vi "ScanDelay_FTIR_BBnorm_Aligning.vi"() -> ()   [LabVIEW 2021]
uses:
  Control_scanDelayWorkflow.ctl
  Control_GetSpectrum_BBnorm.ctl
  C:/Users/mnopl/Desktop/Software/mnOPSuite/PRISM/Thorlabs.MotionControl.FilterFlipperCLI.dll
  Thorlabs.MotionControl.FilterFlipperCLI.dll
  C:/Users/mnopl/Desktop/Software/mnOPSuite/PRISM/Thorlabs.MotionControl.Controls.dll
  Thorlabs.MotionControl.Controls.dll
panel:
  in  "Realign phase":bool
  in  "Recalibrate BB\nfrequency":bool
  in  "Pause\nacquisition":bool
  in  "Replicate\nfrom #":i8=2 min=0
  in  "Envelope width":dbl(slide)=1.0454545454545454 scale=0.25..4.0
  out "Accumulated sample BB spectrum":dbl[][](array[numeric])
  out "Accumulated sample spectrum":dbl[][](array[numeric])
  in  "BB-reference spectrum":bool
  in  "Acquire only\nBB 100% curve with spoofed flip":bool
  in  "Acquire only\nBB 100% curve":bool
  in  "Toggle pause (ms)":dbl=500.0
  out "BB-referenced spectrum (phase)":T1(graph)
  out "BB-referenced spectrum (amplitude)":T2(graph)
  out "Reference BB spectra":dbl[][](array[numeric])
  out "Reference spectra":dbl[][](array[numeric])
  out "Latest replication cmd":string="@rep load 2"
  in  "Replicate\nalpha on\naccumulation":bool=TRUE
  out "# Accumulated":i32
  in  "Accumulate to #":i32=10
  in  "Cancel\nacquisition":bool
  out "Toggle position":i32=1
  in  "BB flipper serial #":string="37005305"
  in  "FilterFlipperControl":refnum<k24>(container)
  out "Spectrum stored":bool
  out "Reference stored":bool=TRUE
  out "Normalized spectrum (phase)":T1(graph)
  out "Normalized spectrum (amplitude)":T1(graph)
  in  "Store as reference":bool
  out "Python alpha rep path":path=path "C:/Users/mnopl/Desktop/Software/python/alpha/rep.py"
  out "Activity status":string="Awaiting command"
  out "Acquisition status":string="Ready to acquire spectrum"
  in  "Path to save spectrum":path=path "C:/Users/mnopl/Desktop/Software/LabVIEW/ScanDelay/Test Data/Ref spectra - silicon 1.txt"
  in  "Load reference":bool
  in  "Path to load reference":path=path "C:/Users/mnopl/Desktop/Software/LabVIEW/ScanDelay/Test Data/Ref spectra - silicon 1.txt"
  in  "Path to load spectrum":path=path "C:/Users/mnopl/Desktop/Software/LabVIEW/ScanDelay/Test Data/Sample spectra - sio2 100 nm.txt"
  in  "Apply spectral\nenvelope":bool=TRUE
  out "Binned interferogram":cluster{"X":dbl, "Y":dbl}[](graph)
  out "Sample BB Spectra":dbl[][](array[numeric])
  out "Sample Spectra":dbl[][](array[numeric])
  out "Python error: spectrum acquisition":errorcluster
  out "Python scandelay path":path=path "C:/Users/mnopl/Desktop/Software/LabVIEW/ScanDelay/scandelay.py"
  in  "Time per\nacquisition (s)":dbl=0.235
  in  "Sampling rate":dbl=250000.0
  in  "Delay calibratior\nfactor (ps/V)":dbl=2.403 format="%_6g"
  in  "Cycles per\ninterferogram":i32=80
  out "Python error: DAQ acquisition":errorcluster
  out "Accumulated spectrum (amplitude)":T3(graph)
  out "Acquisition cycle":dbl[][](graph)
  out "% averaged":dbl=100.0
  in  "Halt program":bool=TRUE
  out "Python error: activity loop":errorcluster
  in  "Load spectrum":bool
  in  "Save spectrum":bool
  in  "Normalize spectrum":bool
  in  "Acquire spectrum":bool
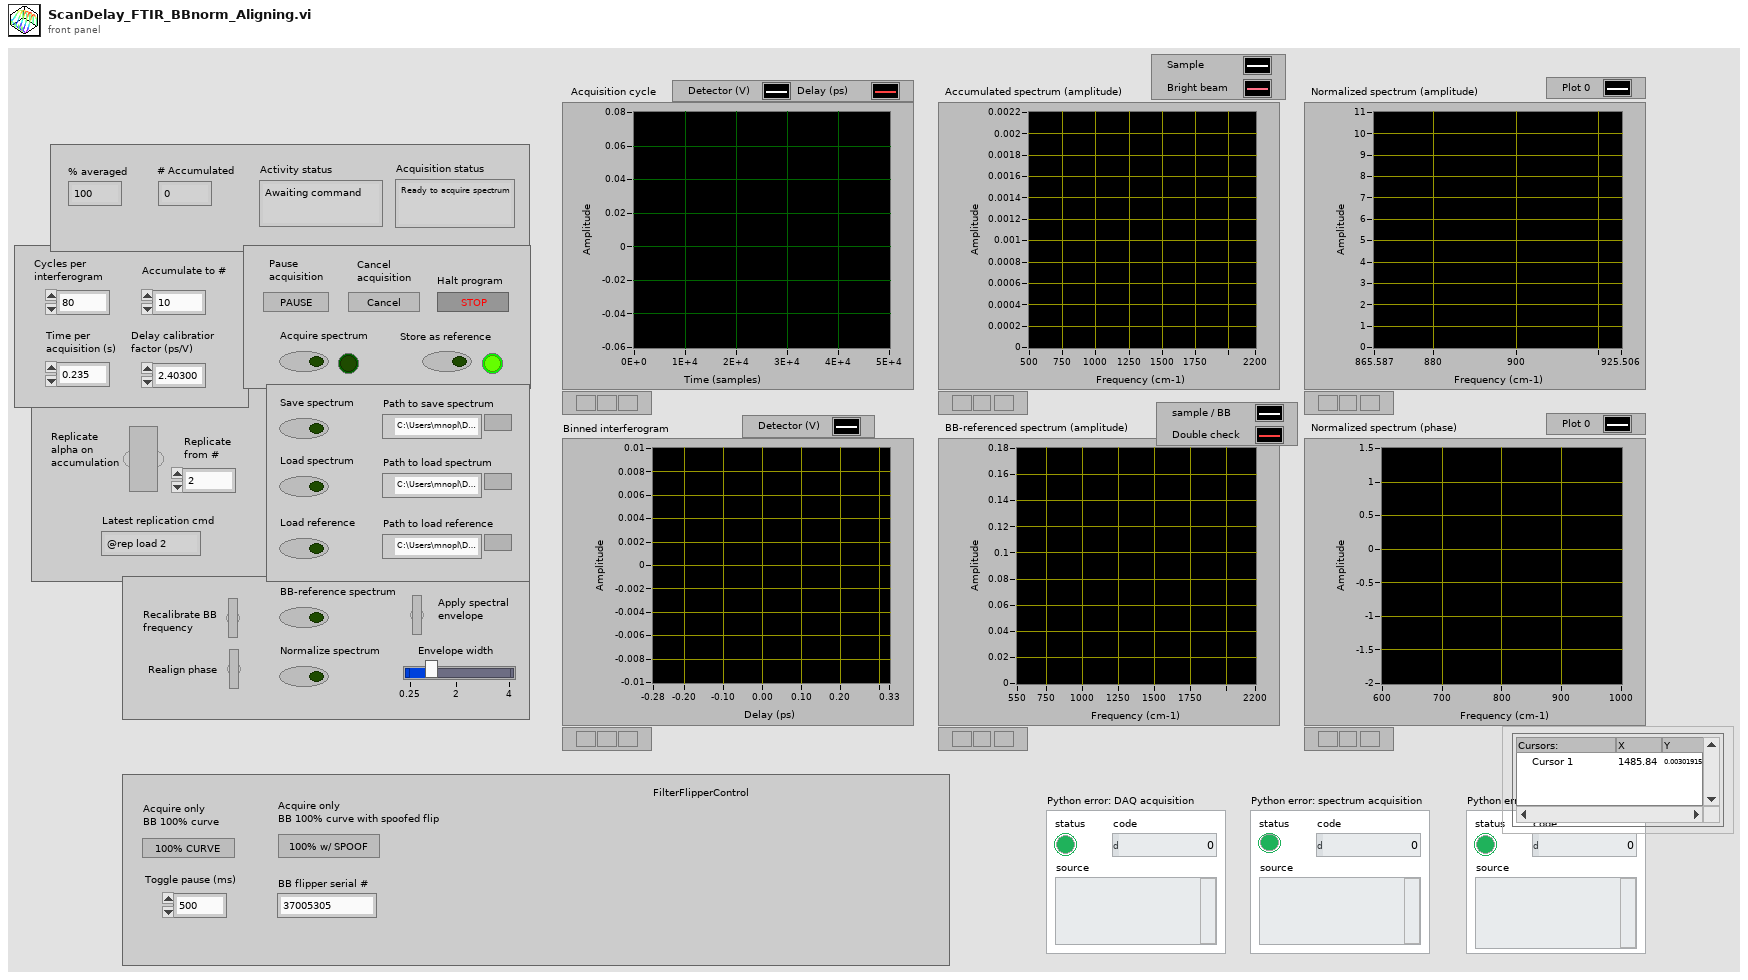
[diagram p1: front panel]
types:
  T1 = cluster{"Output spectrum":dbl[], "Output spectrum":dbl[]}
  T2 = cluster{"Sample Spectra":dbl[], "Sample Spectra":dbl[]}
  T3 = cluster{"Output spectrum":dbl[], "Output spectrum":dbl[]}[]
  T4 = typedef "Control_scanDelayWorkflow.ctl" = enum16{"Initialize", "Sit Idle", "Load Spectrum", "Store reference", "Save Spectrum", "Load reference", "Check Reference", "Check Spectrum", "BB reference spectrum", "Normalize Spectrum", "Done"}
  T5 = typedef "Control_GetSpectrum_BBnorm.ctl" = enum16{"Initialize", "Replicate alpha", "Flip in BB", "Get Spectrum", "Accumulate BB spectrum", "Flip out BB", "Accumulate sample spectrum", "Assess accumulation", "Finalize", "Done"}
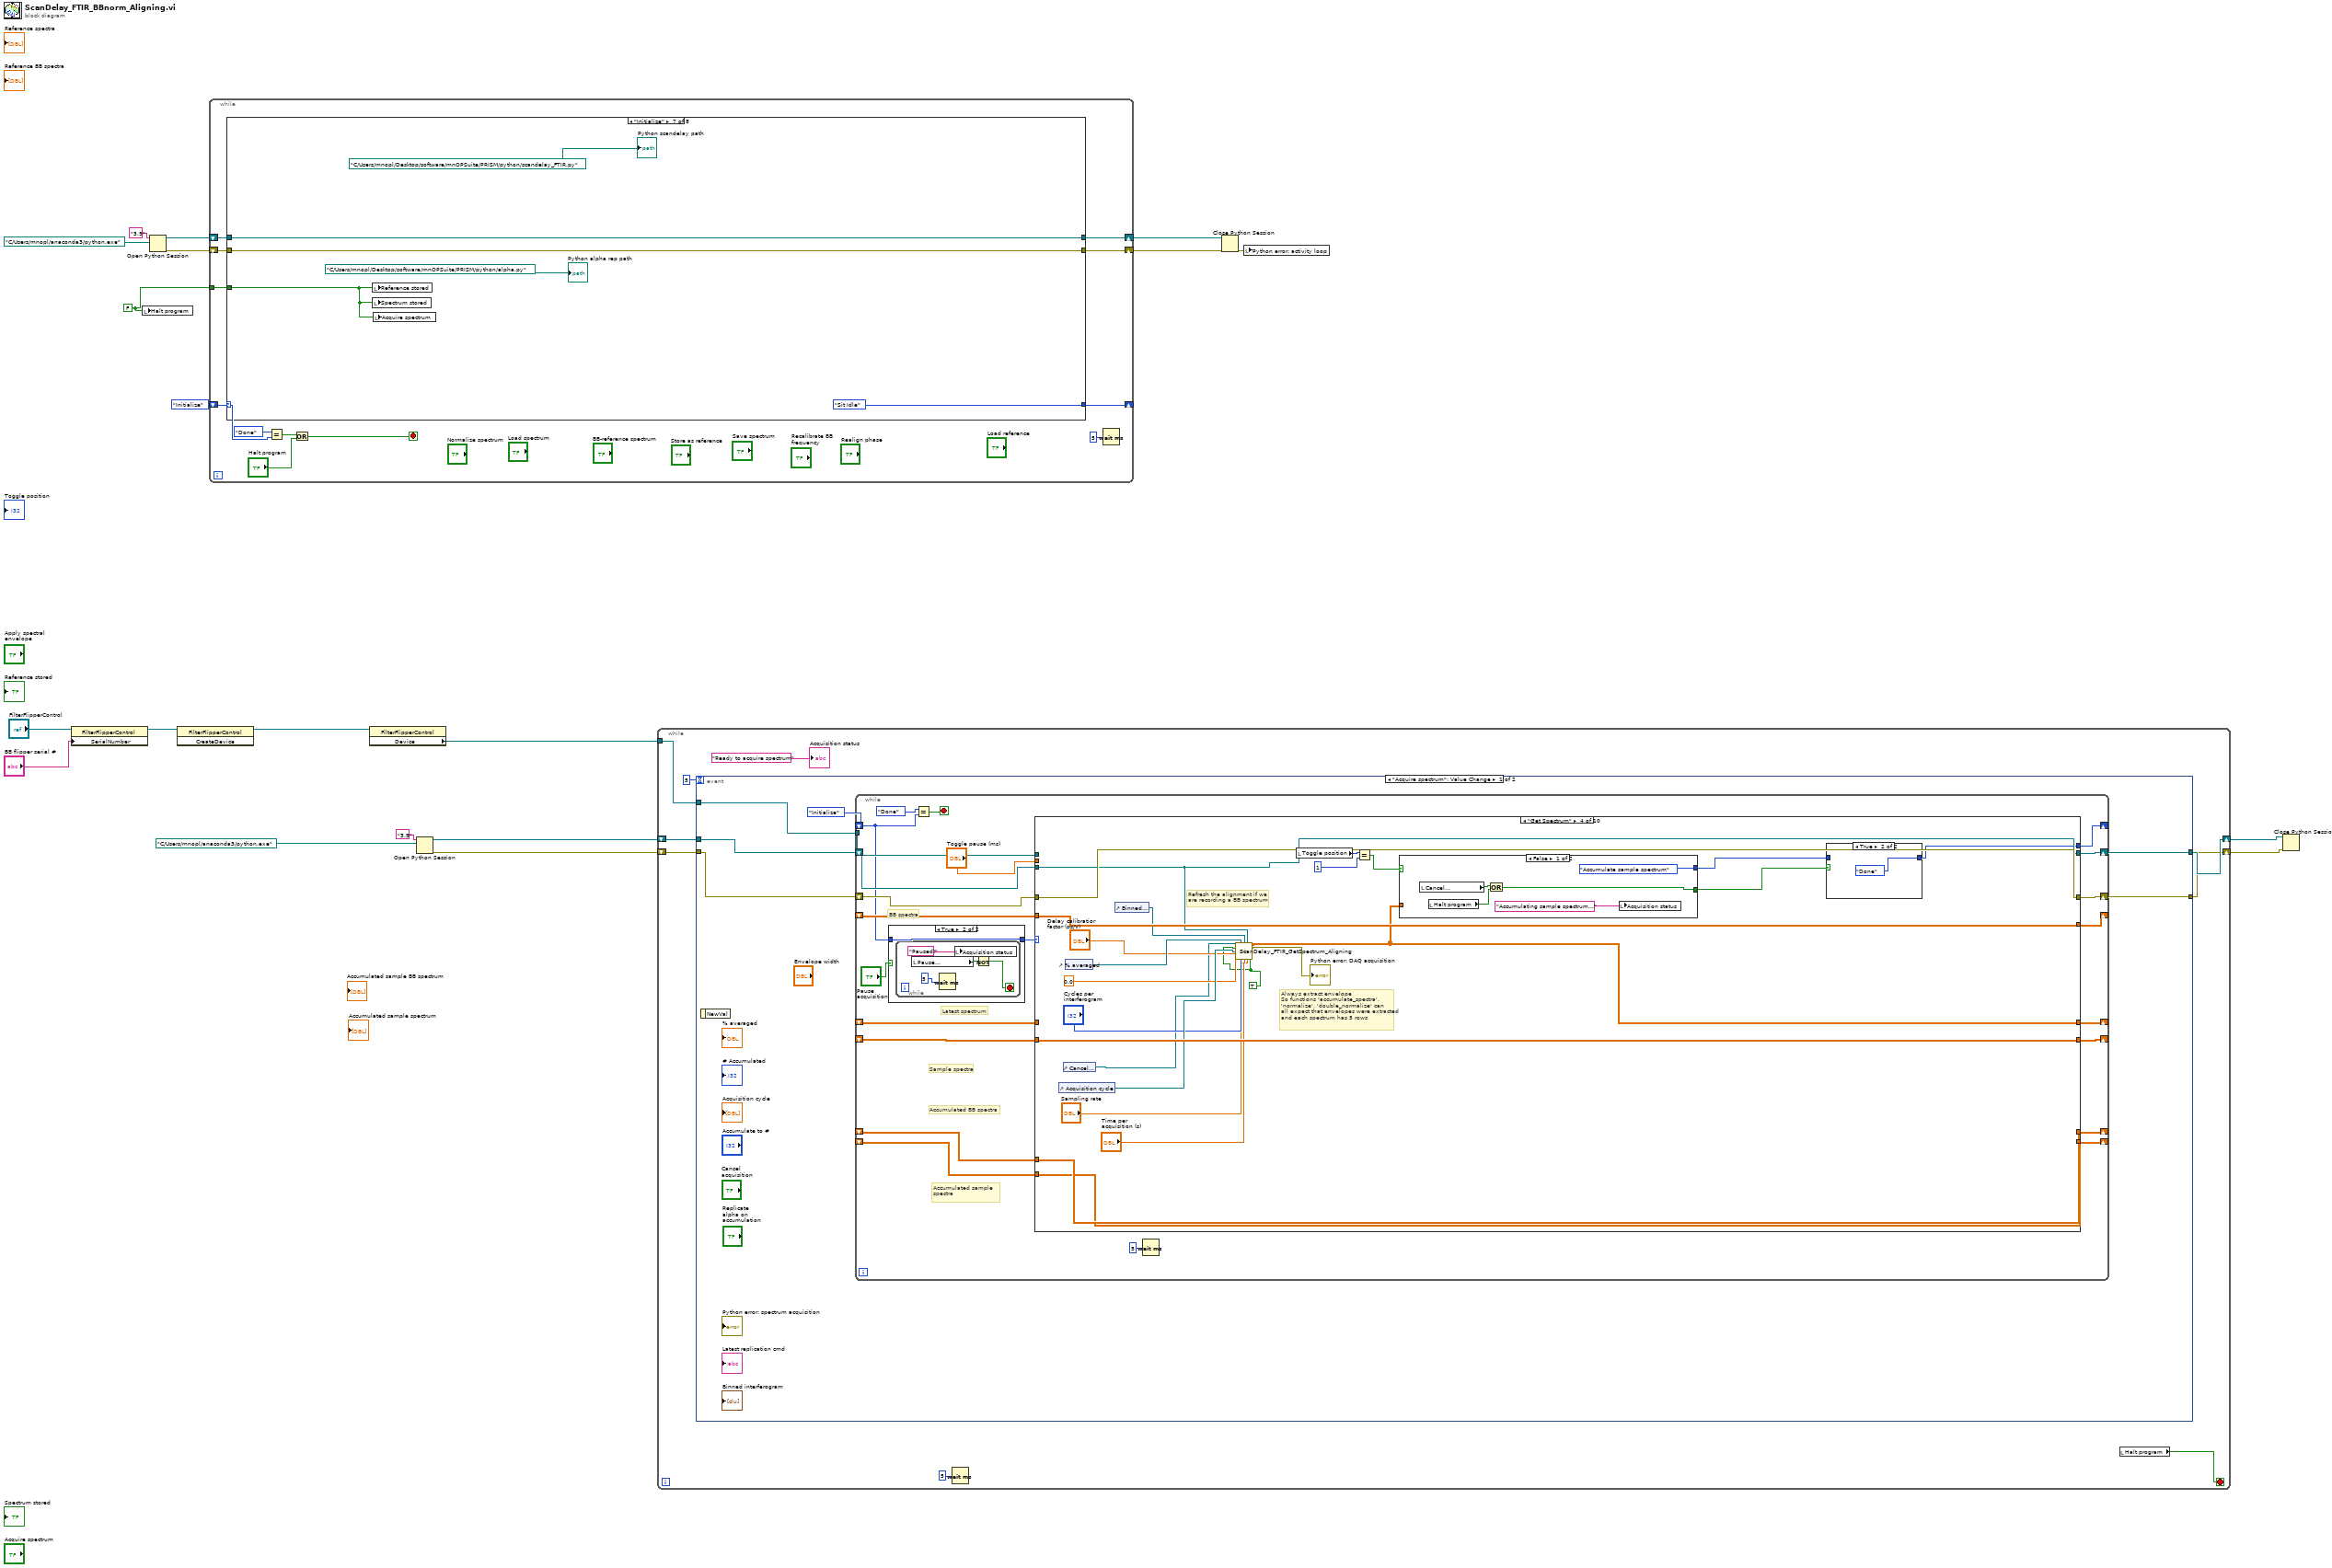
[diagram p0: block diagram]
diagram:
  w1 = FALSE
  n1 = property class="FilterFlipperControl"(reference="FilterFlipperControl", "SerialNumber"="BB flipper serial #") -> (reference out=w11:refnum<k24>)  [unwired: 1 in, 1 out]
  n2 = local write "Halt program"(w1) -> ()
  n3 = Open Python Session(python version="3.9", python path=path "C:/Users/mnopl/anaconda3/python.exe") -> (session out=w16:refnum<k35>, error out=w15:errorcluster)  [unwired: 1 in]
  n4 = invoke class="FilterFlipperControl" method="CreateDevice"(reference=w11) -> (reference out=w10:refnum<k24>)  [unwired: 2 in, 2 out]
  n5 = while {
    shift-right: [w25] -> _
    shift-left: Control_scanDelayWorkflow."Initialize" -> [w22]
    shift-right: [w31] -> w17
    shift-left: w15 -> [w23]
    shift-right: [w26] -> w18
    shift-left: w16 -> [w24]
    tunnel: w1 -> [w21]
    stop <- w29 stop-if-true
    n6 = case shown="\"Initialize\"" w22 {
      tunnel: [w36 w70 w80 w99 w120 w165 w184 w196] -> w31
      tunnel: w24 -> [w37 w69 w79 w100 w123 w166 w185 w194]
      tunnel: w23 -> [w36 w70 w80 w99 w122 w165 w184 w193]
      tunnel: [w37 w69 w79 w100 w121 w166 w185 w195] -> w26
      tunnel: [w35 Control_scanDelayWorkflow."Sit Idle" Control_scanDelayWorkflow."Sit Idle" Control_scanDelayWorkflow."Sit Idle" Control_scanDelayWorkflow."Sit Idle" Control_scanDelayWorkflow."Sit Idle" Control_scanDelayWorkflow."Sit Idle" Control_scanDelayWorkflow."Sit Idle"] -> w25
      tunnel: w21 -> [_ _ _ _ _ _ w181 _]
      frame "Sit Idle", Default {
        n7 = event shown="[2] \"BB-reference spectrum\": Value Change" {
          selector: _ -> [_ _ _ _ _ _ _]
          dyn-events: _ -> [_ _ _ _ _ _ _]
          timeout: 5 -> [_ _ _ _ _ _ w62]
          tunnel: [w38 w42 w49 w50 w54 w58 Control_scanDelayWorkflow."Sit Idle"] -> w35
          event "Normalize spectrum": Value Change {
            n8 = event-data() -> ("NewVal"=w39:bool)  [unwired: 1 in]
            n9 = Select(t=Control_scanDelayWorkflow."Normalize Spectrum", s=w39, f=Control_scanDelayWorkflow."Sit Idle") -> (s? t:f=w38:T4)
          }
          event "Store as reference": Value Change {
            n10 = event-data() -> ("NewVal"=w45:bool)  [unwired: 1 in]
            n11 = Select(t=Control_scanDelayWorkflow."Store reference", s=w45, f=Control_scanDelayWorkflow."Sit Idle") -> (s? t:f=w42:T4)
          }
          event "BB-reference spectrum": Value Change {
            n12 = event-data() -> ("NewVal"=w47:bool)  [unwired: 1 in]
            n13 = Select(t=Control_scanDelayWorkflow."BB reference spectrum", s=w47, f=Control_scanDelayWorkflow."Sit Idle") -> (s? t:f=w49:T4)
          }
          event "Save spectrum": Value Change {
            n14 = event-data() -> ("NewVal"=w51:bool)  [unwired: 1 in]
            n15 = Select(t=Control_scanDelayWorkflow."Save Spectrum", s=w51, f=Control_scanDelayWorkflow."Sit Idle") -> (s? t:f=w50:T4)
          }
          event "Load reference": Value Change {
            n16 = event-data() -> ("NewVal"=w57:bool)  [unwired: 1 in]
            n17 = Select(t=Control_scanDelayWorkflow."Load reference", s=w57, f=Control_scanDelayWorkflow."Sit Idle") -> (s? t:f=w54:T4)
          }
          event "Load spectrum": Value Change {
            n18 = event-data() -> ("NewVal"=w59:bool)  [unwired: 1 in]
            n19 = Select(t=Control_scanDelayWorkflow."Load Spectrum", s=w59, f=Control_scanDelayWorkflow."Sit Idle") -> (s? t:f=w58:T4)
          }
          event Timeout {
            n20 = event-data() -> ()  [unwired: 1 in, 2 out]
            n21 = Wait (ms)(milliseconds to wait=w62) -> ()  [unwired: 1 out]
          }
        }
        "Activity status" <- "Awaiting command"
      }
      frame "Store reference" {
        # "Is spectrum a full array?"
        n22 = local read "Sample Spectra"() -> (w65:dbl[][])
        n23 = local read "Sample BB Spectra"() -> (w64:dbl[][])
        n24 = Empty Array?(array=w65) -> (empty?=w67:bool)
        n25 = Not(x=w67) -> (.not. x?=w66:bool)
        n26 = case shown="True" w66 {
          tunnel: w65 -> [_ w73]
          tunnel: w64 -> [_ w74]
          frame False {
            n27 = Wait (ms)(milliseconds to wait=1000) -> ()  [unwired: 1 out]
            n28 = local write "Activity status"("Error: Spectrum is empty!") -> ()
          }
          frame True {
            n29 = local write "Reference BB spectra"(w74) -> ()
            n30 = local write "Reference spectra"(w73) -> ()
            n31 = local write "Reference stored"(TRUE) -> ()
            n32 = Wait (ms)(milliseconds to wait=1000) -> ()  [unwired: 1 out]
            n33 = local write "Activity status"("Storing reference!") -> ()
          }
        }
      }
      frame "Save Spectrum" {
        n34 = flat-sequence {
          frame #0 {
            w86 = "%g"
            n35 = local read "Sample Spectra"() -> (w88:dbl[][])
            n36 = Path To String(path="Path to save spectrum") -> (string=w90:string)
            n37 = local read "Sample BB Spectra"() -> (w81:dbl[][])
            n38 = Search and Replace String(input string=w90, search string="(.txt)*$", replace string=".txt") -> (result string=w94:string)  [unwired: 5 in, 3 out]
            n39 = Search and Replace String(input string=w94, search string=".txt$", replace string="_BB.txt") -> (result string=w93:string)  [unwired: 5 in, 3 out]
            n40 = String To Path(string=w94) -> (path=w91:path)
            n41 = Array To Spreadsheet String(array=w88, 3:w86) -> (spreadsheet string=w87:string)  [unwired: 1 in]
            n42 = Array To Spreadsheet String(array=w81, 3:w86) -> (spreadsheet string=w95:string)  [unwired: 1 in]
            n43 = String To Path(string=w93) -> (path=w92:path)
            n44 = Write to Text File(file (use dialog)=w91, text=w87) -> ()  [unwired: 2 in, 3 out]
            n45 = Write to Text File(file (use dialog)=w92, text=w95) -> ()  [unwired: 2 in, 3 out]
          }
          frame #1 {
            n46 = local write "Activity status"("Successfully saved spectrum!") -> ()
            n47 = Wait (ms)(milliseconds to wait=1000) -> ()  [unwired: 1 out]
          }
        }
      }
      frame "Load reference" {
        n48 = flat-sequence {
          frame #0 {
            w105 = "%g"
            n49 = Path To String(path="Path to load reference") -> (string=w101:string)
            n50 = Search and Replace String(input string=w101, search string=".txt$", replace string="_BB.txt") -> (result string=w103:string)  [unwired: 5 in, 3 out]
            n51 = Read from Text File(file (use dialog)="Path to load reference") -> (text=w106:string)  [unwired: 3 in, 3 out]
            n52 = String To Path(string=w103) -> (path=w110:path)
            n53 = Spreadsheet String To Array(format string=w105, spreadsheet string=w106) -> (array=w107:dbl[][])  [unwired: 2 in]
            n54 = Read from Text File(file (use dialog)=w110) -> (text=w109:string)  [unwired: 3 in, 3 out]
            n55 = local write "Reference spectra"(w107) -> ()
            n56 = Spreadsheet String To Array(format string=w105, spreadsheet string=w109) -> (array=w111:dbl[][])  [unwired: 2 in]
            n57 = local write "Reference BB spectra"(w111) -> ()
          }
          frame #1 {
            n58 = local write "Reference stored"(TRUE) -> ()
            n59 = Wait (ms)(milliseconds to wait=1000) -> ()  [unwired: 1 out]
            n60 = local write "Activity status"("Successfully loaded reference!") -> ()
          }
        }
      }
      frame "Normalize Spectrum" {
        n61 = local read "Reference stored"() -> (w117:bool)
        n62 = local read "Spectrum stored"() -> (w116:bool)
        n63 = And(x=w116, y=w117) -> (x .and. y?=w115:bool)
        n64 = flat-sequence {
          tunnel: w123 -> [w129]
          tunnel: w122 -> [w128]
          tunnel: [w127] -> w119
          tunnel: [w126] -> w118
          tunnel: w115 -> [w125]
          tunnel: [w162] -> w120
          tunnel: [w163] -> w121
          tunnel: w119 -> [w163]
          tunnel: w118 -> [w162]
          frame #0 {
            n65 = case shown="True" w125 {
              tunnel: w129 -> [w131 w159]
              tunnel: w128 -> [w130 w158]
              tunnel: [w131 w157] -> w127
              tunnel: [w130 w140] -> w126
              frame False {
                n66 = Wait (ms)(milliseconds to wait=1000) -> ()  [unwired: 1 out]
                n67 = local write "Activity status"("Error: Spectrum or reference is empty!") -> ()
              }
              frame True {
                n68 = Wait (ms)(milliseconds to wait=1000) -> ()  [unwired: 1 out]
                n69 = local read "Python scandelay path"() -> (w156:path)
                n70 = local read "Sample Spectra"() -> (w141:dbl[][])
                n71 = local read "Sample BB Spectra"() -> (w142:dbl[][])
                n72 = local read "Reference spectra"() -> (w139:dbl[][])
                n73 = local read "Reference BB spectra"() -> (w138:dbl[][])
                n74 = local read "Apply spectral\nenvelope"() -> (w137:bool)
                n75 = local read "Envelope width"() -> (w136:dbl)
                n76 = local read "Recalibrate BB\nfrequency"() -> (w135:bool)
                n77 = local read "Realign phase"() -> (w134:bool)
                n78 = local write "Activity status"("Normalizing spectrum!") -> ()
                n79 = node(w159, w156, "normalized_spectrum", w158, w141, w141, w142, w139, w138, w137, w136, w135, w134) -> (w157:refnum<k35>, w140:errorcluster, w144:dbl[][])  [unwired: 8 in, 2 out]
                "Python error: activity loop" <- w140
                n80 = Index Array(array=w144, index (row) #1=0, index (row) #2=1) -> (element #1=w152:dbl[], element #2=w151:dbl[])  [unwired: 2 in]
                n81 = Index Array(array=w144, index (row) #1=0, index (row) #2=2) -> (element #1=w148:dbl[], element #2=w147:dbl[])  [unwired: 2 in]
                n82 = Bundle("Sample Spectra"=w152, "Sample Spectra"=w151) -> (→"Normalized spectrum (amplitude)":T2)  [unwired: 1 in]
                n83 = Bundle("Sample Spectra"=w148, "Sample Spectra"=w147) -> (→"Normalized spectrum (phase)":T2)  [unwired: 1 in]
              }
            }
          }
          frame #1 {
            n84 = local write "Normalize spectrum"(FALSE) -> ()
          }
        }
      }
      frame "Load Spectrum" {
        n85 = flat-sequence {
          frame #0 {
            w174 = "%g"
            n86 = Path To String(path="Path to load spectrum") -> (string=w170:string)
            n87 = Search and Replace String(input string=w170, search string=".txt$", replace string="_BB.txt") -> (result string=w172:string)  [unwired: 5 in, 3 out]
            n88 = Read from Text File(file (use dialog)="Path to load spectrum") -> (text=w175:string)  [unwired: 3 in, 3 out]
            n89 = String To Path(string=w172) -> (path=w177:path)
            n90 = Spreadsheet String To Array(format string=w174, spreadsheet string=w175) -> (array=w168:dbl[][])  [unwired: 2 in]
            n91 = Read from Text File(file (use dialog)=w177) -> (text=w176:string)  [unwired: 3 in, 3 out]
            n92 = Spreadsheet String To Array(format string=w174, spreadsheet string=w176) -> (array=w167:dbl[][])  [unwired: 2 in]
            n93 = local write "Sample Spectra"(w168) -> ()
            n94 = local write "Sample BB Spectra"(w167) -> ()
          }
          frame #1 {
            n95 = local write "Spectrum stored"(TRUE) -> ()
            n96 = local write "Activity status"("Successfully loaded spectrum!") -> ()
            n97 = Wait (ms)(milliseconds to wait=1000) -> ()  [unwired: 1 out]
          }
        }
      }
      frame "Initialize" {
        n98 = local write "Reference stored"(w181) -> ()
        n99 = local write "Spectrum stored"(w181) -> ()
        n100 = local write "Acquire spectrum"(w181) -> ()
        "Python scandelay path" <- path "C:/Users/mnopl/Desktop/software/mnOPSuite/PRISM/python/scandelay_FTIR.py"
        "Python alpha rep path" <- path "C:/Users/mnopl/Desktop/software/mnOPSuite/PRISM/python/alpha.py"
      }
      frame "BB reference spectrum" {
        # "Is spectrum a full array?"
        n101 = local read "Sample Spectra"() -> (w187:dbl[][])
        n102 = Empty Array?(array=w187) -> (empty?=w189:bool)
        n103 = Not(x=w189) -> (.not. x?=w188:bool)
        n104 = flat-sequence {
          tunnel: w194 -> [w200]
          tunnel: w193 -> [w199]
          tunnel: w188 -> [w198]
          tunnel: [w202] -> w191
          tunnel: [w201] -> w190
          tunnel: w187 -> [w197]
          tunnel: [w233] -> w195
          tunnel: [w234] -> w196
          tunnel: w191 -> [w234]
          tunnel: w190 -> [w233]
          frame #0 {
            n105 = case shown="True" w198 {
              tunnel: [w203 w211] -> w202
              tunnel: [w204 w212] -> w201
              tunnel: w200 -> [w204 w221]
              tunnel: w199 -> [w203 w220]
              tunnel: w197 -> [_ w216]
              frame False {
                n106 = Wait (ms)(milliseconds to wait=1000) -> ()  [unwired: 1 out]
                n107 = local write "Activity status"("Error: Spectrum or reference is empty!") -> ()
              }
              frame True {
                n108 = local read "Python scandelay path"() -> (w215:path)
                n109 = local read "Sample BB Spectra"() -> (w219:dbl[][])
                n110 = local read "Apply spectral\nenvelope"() -> (w210:bool)
                n111 = local read "Envelope width"() -> (w209:dbl)
                n112 = local read "Recalibrate BB\nfrequency"() -> (w208:bool)
                n113 = local read "Realign phase"() -> (w207:bool)
                n114 = Wait (ms)(milliseconds to wait=1000) -> ()  [unwired: 1 out]
                n115 = local write "Activity status"("Referencing spectrum to bright beam...") -> ()
                n116 = node(w221, w215, "BB_referenced_spectrum", w220, w216, w216, w219, w210, w209, w208, w207) -> (w212:refnum<k35>, w211:errorcluster, w226:dbl[][])  [unwired: 6 in, 2 out]
                n117 = local write "Python error: activity loop"(w211) -> ()
                n118 = Index Array(array=w226, index (row) #1=0, index (row) #2=2) -> (element #1=w229:dbl[], element #2=w228:dbl[])  [unwired: 2 in]
                n119 = Index Array(array=w226, index (row) #1=0, index (row) #2=1) -> (element #1=w231:dbl[], element #2=w230:dbl[])  [unwired: 2 in]
                n120 = Bundle("Sample Spectra"=w229, "Sample Spectra"=w228) -> (→"BB-referenced spectrum (phase)":T2)  [unwired: 1 in]
                n121 = Bundle("Sample Spectra"=w231, "Sample Spectra"=w230) -> (→"BB-referenced spectrum (amplitude)":T2)  [unwired: 1 in]
              }
            }
          }
          frame #1 {
            n122 = local write "BB-reference spectrum"(FALSE) -> ()
          }
        }
      }
    }
    n123 = Equal?(x=Control_scanDelayWorkflow."Done", y=w22) -> (x = y?=w27:bool)
    n124 = Or(x=w27, y="Halt program") -> (x .or. y?=w29:bool)
    n125 = Wait (ms)(milliseconds to wait=5) -> ()  [unwired: 1 out]
  }
  n126 = property class="FilterFlipperControl"(reference=w10) -> ("Device"=w4:refnum<k24>)  [unwired: 1 in, 2 out]
  n127 = Open Python Session(python version="3.9", python path=path "C:/Users/mnopl/anaconda3/python.exe") -> (session out=w6:refnum<k35>, error out=w5:errorcluster)  [unwired: 1 in]
  n128 = while {
    tunnel: w4 -> [w237]
    shift-right: [w235] -> w2
    shift-left: w5 -> [w238]
    shift-right: [w236] -> w3
    shift-left: w6 -> [w239]
    stop <- w243 stop-if-true
    n129 = event shown="[0] \"Acquire spectrum\": Value Change" {
      selector: _ -> [_ _]
      dyn-events: _ -> [_ _]
      timeout: 5 -> [_ w500]
      tunnel: w239 -> [w248 w499]
      tunnel: w238 -> [w247 w498]
      tunnel: w237 -> [w246 _]
      tunnel: [w245 w499] -> w236
      tunnel: [w244 w498] -> w235
      event "Acquire spectrum": Value Change {
        n130 = event-data() -> ()  [unwired: 1 in, 1 out]
        n131 = while {
          shift-right: [w270] -> _
          shift-left: _ -> [w269]
          shift-right: [w271] -> _
          shift-left: _ -> [w268]
          shift-right: [w267] -> _
          shift-left: Control_GetSpectrum_BBnorm."Initialize" -> [w252]
          shift-right: [w264] -> w244
          shift-left: w247 -> [w265]
          shift-right: [w263] -> w245
          shift-left: w248 -> [w266]
          shift-right: [w262] -> _
          shift-left: _ -> [w260]
          tunnel: w246 -> [w259]
          shift-right: [w257] -> _
          shift-left: _ -> [w255]
          shift-right: [w256] -> _
          shift-left: _ -> [w254]
          stop <- w250 stop-if-true
          # "BB spectra"
          # "Accumulated BB spectra"
          # "Accumulated sample spectra"
          # "Sample spectra"
          # "Latest spectrum"
          n132 = case shown="True" "Pause\nacquisition" {
            tunnel: w252 -> [w273 w274]
            tunnel: [w273 w274] -> w251
            frame False {
            }
            frame True {
              n133 = while {
                stop <- w278 stop-if-true
                n134 = local read "Pause\nacquisition"() -> (w277:bool)
                n135 = Wait (ms)(milliseconds to wait=5) -> ()  [unwired: 1 out]
                n136 = local write "Acquisition status"("Paused!") -> ()
                n137 = Not(x=w277) -> (.not. x?=w278:bool)
              }
            }
          }
          n138 = Equal?(x=Control_GetSpectrum_BBnorm."Done", y=w252) -> (x = y?=w250:bool)
          n139 = case shown="\"Get Spectrum\"" w251 {
            tunnel: [w279 w307 w314 w347 w369 w407 w433 w455 w482 w493] -> w271
            tunnel: [w279 w308 w315 w346 w382 w408 w426 w456 w481 w495] -> w270
            tunnel: w269 -> [_ w308 w315 w346 w391 w408 w426 w456 w481 w495]
            tunnel: w268 -> [_ w307 w314 w347 w369 w407 w434 w455 w482 w493]
            tunnel: [w286 Control_GetSpectrum_BBnorm."Flip in BB" Control_GetSpectrum_BBnorm."Get Spectrum" w326 w376 Control_GetSpectrum_BBnorm."Get Spectrum" Control_GetSpectrum_BBnorm."Assess accumulation" w458 Control_GetSpectrum_BBnorm."Done" Control_GetSpectrum_BBnorm."Done"] -> w267
            tunnel: w266 -> [w283 w304 w317 w341 w386 w406 w444 w460 w484 w497]
            tunnel: w265 -> [w282 w303 w316 w348 w385 w405 w443 w461 w483 w496]
            tunnel: [w282 w297 w316 w348 w375 w405 w432 w461 w483 w496] -> w264
            tunnel: [w283 w298 w317 w341 w384 w406 w442 w460 w484 w497] -> w263
            tunnel: w259 -> [_ _ w312 _ _ w403 _ _ _ _]
            tunnel: [w279 w296 w313 w331 w377 w404 w436 w457 w488 w494] -> w262
            tunnel: w260 -> [_ w296 w313 _ w377 w404 w436 w457 w488 w494]
            tunnel: "Toggle pause (ms)" -> [_ _ w311 _ _ w402 _ _ _ _]
            tunnel: [w279 w295 w310 w343 w365 w401 w423 w453 w486 w491] -> w257
            tunnel: [w279 w294 w309 w342 w363 w400 w424 w454 w485 w490] -> w256
            tunnel: w255 -> [_ w295 w310 w343 w363 w401 w423 w453 w486 w491]
            tunnel: w254 -> [_ w294 w309 w342 w364 w400 _ w454 w485 w490]
            frame "Initialize", Default {
              w287 = dbl[] []
              n140 = local write "Toggle position"(1) -> ()
              n141 = local write "# Accumulated"(0) -> ()
              n142 = local write "Spectrum stored"(FALSE) -> ()
              n143 = local read "Replicate\nalpha on\naccumulation"() -> (w284:bool)
              n144 = case shown="False" w284 {
                tunnel: [Control_GetSpectrum_BBnorm."Flip in BB" Control_GetSpectrum_BBnorm."Replicate alpha"] -> w286
                frame False {
                }
                frame True {
                  n145 = local write "Acquisition status"("Replicating alpha...") -> ()
                }
              }
              n146 = Build Array(w287, w287) -> (w279:dbl[][])
              "Sample Spectra" <- w279
              "Sample BB Spectra" <- w279
            }
            frame "Replicate alpha" {
              w301 = "replicate"
              # "Wait time for replication (s)"
              n147 = local write "Acquisition status"("Replicating alpha...") -> ()
              n148 = local read "# Accumulated"() -> (w293:i32)
              n149 = Add(x=w293, y="Replicate\nfrom #") -> (x+y=w291:i32)
              n150 = local read "Python alpha rep path"() -> (w302:path)
              n151 = node(w304, w302, w301, w303, w301, w291, 8) -> (w298:refnum<k35>, w297:errorcluster, w299:string)  [unwired: 2 in, 2 out]
              n152 = local write "Python error: spectrum acquisition"(w297) -> ()
              n153 = local write "Latest replication cmd"(w299) -> ()
            }
            frame "Flip in BB" {
              n154 = flat-sequence {
                tunnel: w312 -> [w322]
                tunnel: w311 -> [w323]
                frame #0 {
                  n155 = local write "Acquisition status"("Toggling to bright beam...") -> ()
                }
                frame #1 {
                  w321 = 1
                  n156 = local write "Toggle position"(w321) -> ()
                  n157 = invoke class="FilterFlipper" method="SetPosition"(reference=w322, "position"=w321, "waitTimeout"=20000) -> ()  [unwired: 2 in, 5 out]
                }
                frame #2 {
                  n158 = Wait (ms)(milliseconds to wait=w323) -> ()  [unwired: 1 out]
                  n159 = local write "Acquisition status"("Acquiring bright beam spectrum...") -> ()
                }
              }
            }
            frame "Get Spectrum" {
              w329 = TRUE
              # "Always extract envelope\nSo functions 'accumulate_spectra',\n'normalize', 'double_normalize' can \nall expect that envelopes were extracted\nand each spectrum has 5 rows"
              # "Refresh the alignment if we\nare recording a BB spectrum"
              n160 = control-ref of="Acquisition cycle"() -> (w338:refnum<vi>)
              n161 = control-ref of="Cancel\nacquisition"() -> (w328:refnum<vi>)
              n162 = control-ref of="% averaged"() -> (w339:refnum<vi>)
              n163 = control-ref of="Binned interferogram"() -> (w340:refnum<vi>)
              n164 = call "ScanDelay_FTIR_GetSpectrum_Aligning.vi"("Cancel? External"=w328, "% averaged (external)"=w339, "Binned interferogram (external)"=w340, "Python refnum in"=w341, "Refresh alignment"=w329, "Acquisition cycle (external)"=w338, "Delay calibration\n          factor"="Delay calibratior\nfactor (ps/V)", "Subtract\ndelay (ps)"=0.0, "Acquisitions per interferogram"="Cycles per\ninterferogram", "Time per\nacquisition (s)"="Time per\nacquisition (s)", "Sampling rate"="Sampling rate", "Extract envelope"=w329) -> ("Output spectrum"=w331:dbl[][], "Python error out"=→"Python error: DAQ acquisition":errorcluster)  [unwired: 2 in]
              n165 = local read "Toggle position"() -> (w345:i32)
              n166 = Equal?(x=w345, y=1) -> (x = y?=w330:bool)
              n167 = case shown="False" w330 {
                tunnel: [Control_GetSpectrum_BBnorm."Accumulate sample spectrum" Control_GetSpectrum_BBnorm."Accumulate BB spectrum"] -> w327
                tunnel: w331 -> [_ _]
                tunnel: [w351 w356] -> w325
                frame False {
                  n168 = local read "Cancel\nacquisition"() -> (w352:bool)
                  n169 = local read "Halt program"() -> (w353:bool)
                  n170 = Or(x=w352, y=w353) -> (x .or. y?=w351:bool)
                  n171 = local write "Acquisition status"("Accumulating sample spectrum...") -> ()
                }
                frame True {
                  n172 = local read "Cancel\nacquisition"() -> (w358:bool)
                  n173 = local read "Halt program"() -> (w357:bool)
                  n174 = Or(x=w358, y=w357) -> (x .or. y?=w356:bool)
                  n175 = local write "Acquisition status"("Accumulating bright beam spectrum...") -> ()
                }
              }
              n176 = case shown="True" w325 {
                tunnel: w327 -> [w349 _]
                tunnel: [w349 Control_GetSpectrum_BBnorm."Done"] -> w326
                frame False {
                }
                frame True {
                }
              }
            }
            frame "Accumulate BB spectrum" {
              n177 = local read "# Accumulated"() -> (w390:i32)
              n178 = Equal?(x=w390, y=0) -> (x = y?=w388:bool)
              n179 = case shown="False" w388 {
                tunnel: w377 -> [w397 w399]
                tunnel: w391 -> [w398 _]
                tunnel: [w396 w399] -> w382
                frame False {
                  n180 = Build Array (concatenate)(w398, w397) -> (w396:dbl[][])
                }
                frame True {
                }
              }
              n181 = local read "Apply spectral\nenvelope"() -> (w362:bool)
              n182 = local read "Python scandelay path"() -> (w383:path)
              n183 = local read "Envelope width"() -> (w361:dbl)
              n184 = node(w386, w383, "accumulate_spectra", w385, w382, w382, w362, w361) -> (w384:refnum<k35>, w375:errorcluster, w365:dbl[][])  [unwired: 3 in, 2 out]
              n185 = Index Array(array=w365, index (row) #1=0, index (row) #2=1) -> (element #1=w379:dbl[], element #2=w378:dbl[])  [unwired: 2 in]
              n186 = Index Array(array=w364, index (row) #1=0, index (row) #2=1) -> (element #1=w371:dbl[], element #2=w370:dbl[])  [unwired: 2 in]
              n187 = Bundle("Output spectrum"=w379, "Output spectrum"=w378) -> (w367:T1)  [unwired: 1 in]
              n188 = Bundle("Output spectrum"=w371, "Output spectrum"=w370) -> (w368:T1)  [unwired: 1 in]
              n189 = local write "Python error: spectrum acquisition"(w375) -> ()